vi "Host - FPGA trig export.vi"() -> ()   [LabVIEW 2019]
uses:
  <vilib>/userdefined/High Color/nirio_resource_hc.ctl
  SubVIs/Low-level/TypeDefs/TX trigger config.ctl
  FPGA/SubVIs/Utility/FPGA driver trigger source.ctl
  FPGA/SubVIs/Utility/FPGA driver trigger destination.ctl
  <vilib>/FPGAPlugInAG/PXIe-7902R/niLvFpga_Open_PXIe-7902R.vi
  <vilib>/rvi/interface/common/dynamic/niFpgaDynamicAddResources.vi
  <vilib>/Utility/error.llb/Error Cluster From Error Code.vi
  <vilib>/rvi/errors/niLvFpgaAdjustHostInterfaceError.vi
  <vilib>/FPGAPlugInAG/Dynamic/niLvFpga_Close_Dynamic.vi
  <vilib>/rvi/interface/nirviOpenFPGA/nirviOpenFPGA.xnode
  FPGA Bitfiles/barkhausenmmwave_ReceiveFPGA(3.07_FPGAtrigexport_4ZkiZJGs6ac.lvbitx
  <vilib>/rvi/interface/nirviReadWriteControl/nirviReadWriteControl.xnode
  <vilib>/rvi/interface/nirviCloseFPGA/nirviCloseFPGA.xnode
  NiFpgaLv.dll
  <vilib>/rvi/interface/Simulation/niFpgaSimulationCallBeginRW.vi
  FPGA/SubVIs/Utility/FPGA Utility.lvlib
panel:
  out "error out":T1
  in  "FPGA 2":bool
  in  "FPGA 1":bool
  in  "Trig share":T2(tab)
  in  "Sync module (export)":tag="PXI2Slot2"
  in  "Export PXI trigger":string(combo)="PXI_Trig0"
  in  "Sync module export terminal":string(combo)="PFI0"
  in  "Sync module import terminal":string(combo)="PFI0"
  in  "Import PXI trigger":string(combo)="PXI_Trig0"
  in  "Sync module (import)":tag="PXI2Slot2"
  out "fpga2.recieved PXI triggers":u16
  out "pxi0 ctr":u16
  out "pxi1 ctr":u16
  out "status":string
  in  "Stop Button":bool
  out "fpga2.recieved trigs":u16
  out "fpga1.generated trigs":u16
  in  "fpga1.trig control":bool
  in  "FPGA 2 trig":T3
  in  "FPGA 1 trig":T3
  in  "FPGA 2":T6
  in  "FPGA 1":T6
  # "MASTER"
  # "SLAVE"
  # "no trigger sharing through timing module"
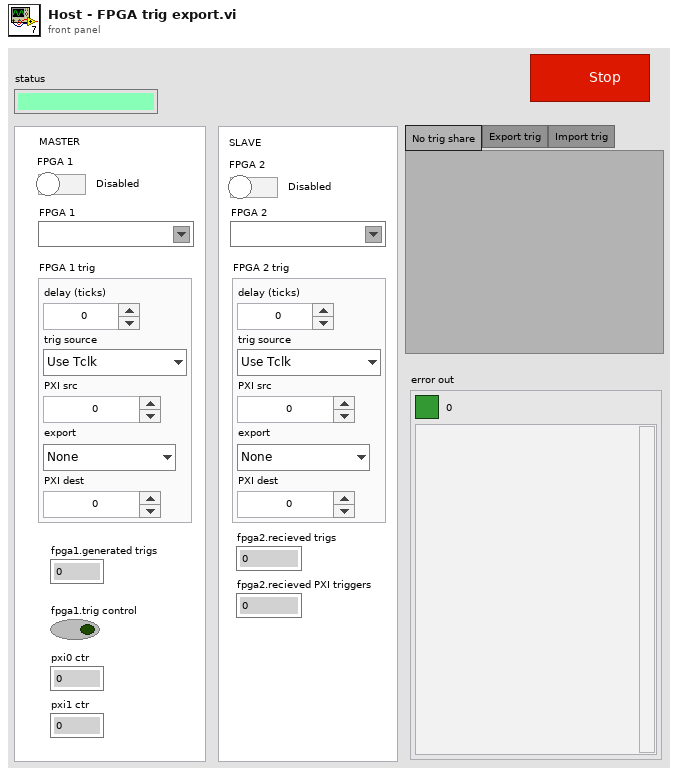
[diagram p1: front panel]
types:
  T1 = cluster{"Boolean Round":bool, "code":i32, "source":string}
  T2 = enum32{"No trig share", "Export trig", "Import trig"}
  T3 = typedef "TX trigger config.ctl" = cluster{"delay (ticks)":u16, "trig source":T4, "PXI src":i32, "export":T5, "PXI dest":i32}
  T4 = typedef "FPGA Utility.lvlib/FPGA driver trigger source.ctl" = enum16{"Use Tclk", "PXI_Trig", "Aurora RX trig"}
  T5 = typedef "FPGA Utility.lvlib/FPGA driver trigger destination.ctl" = enum16{"None", "Source trig", "Synced trig", "Delayed sync"}
  T6 = typedef "nirio_resource_hc.ctl" = tag
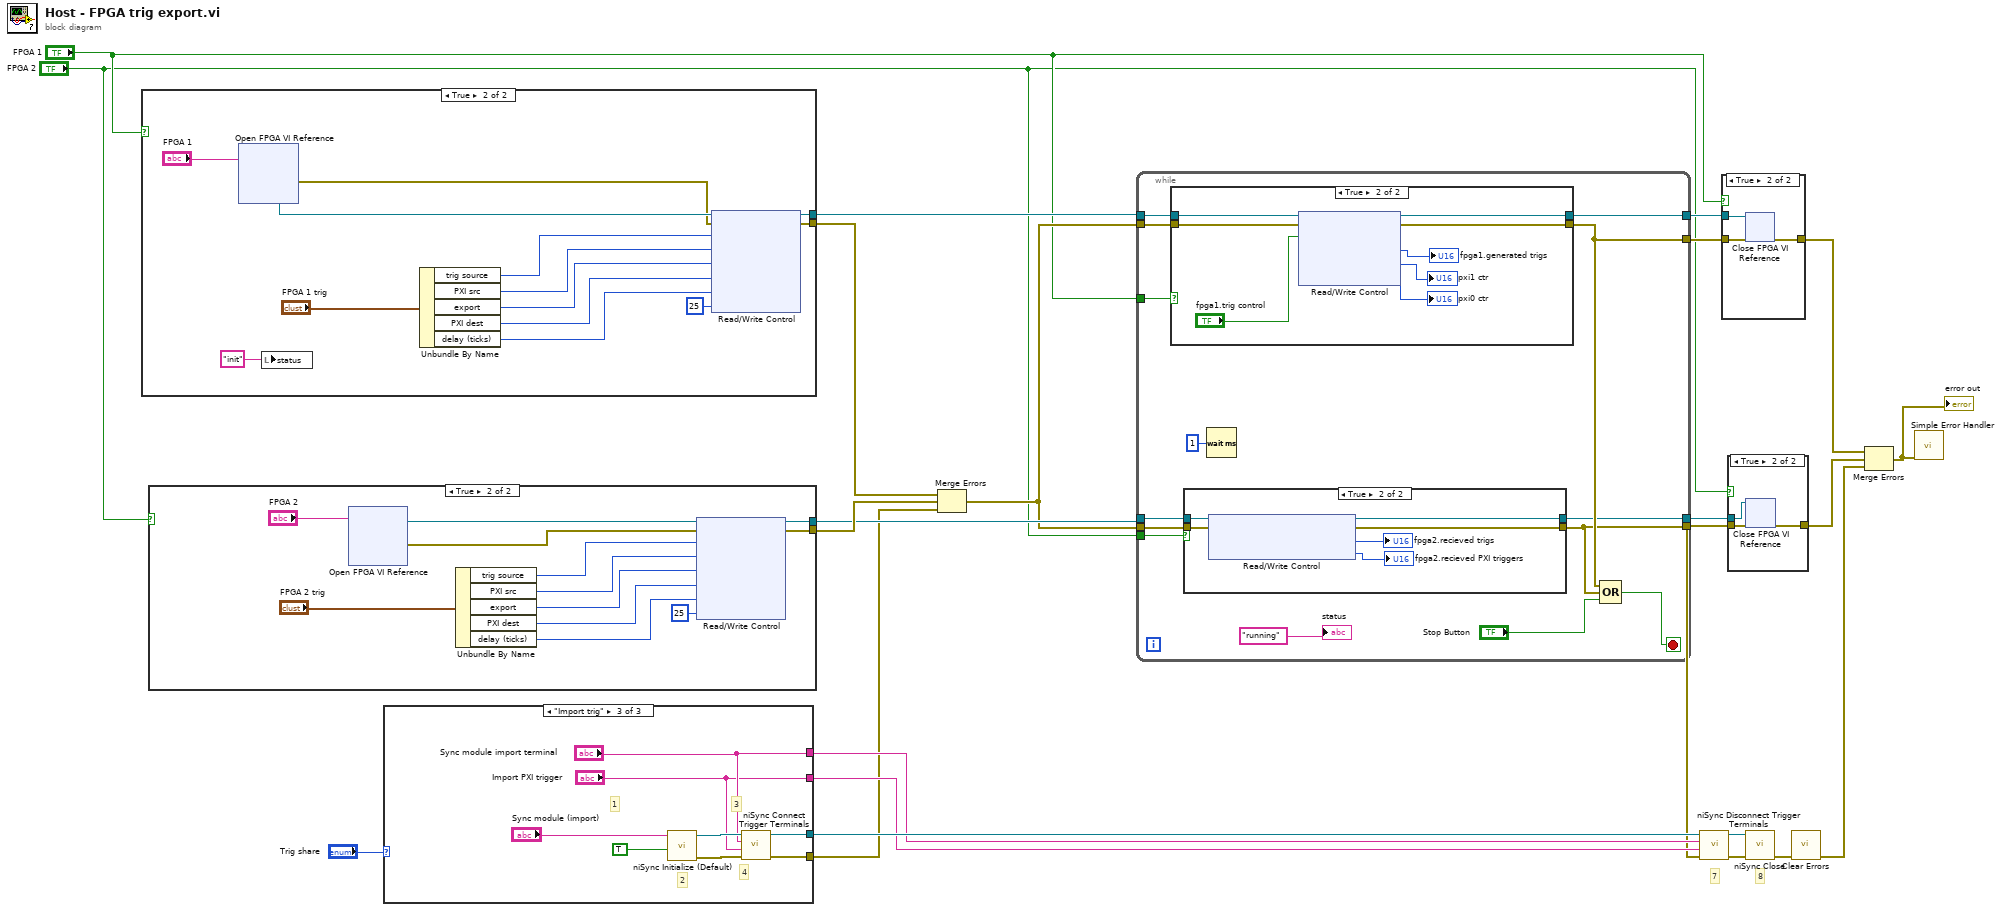
[diagram p0: block diagram]
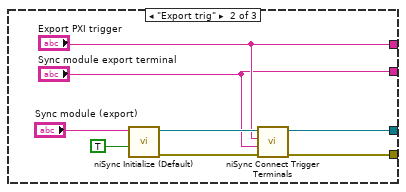
[diagram p7: hidden frame]
diagram:
  # "8"
  # "7"
  n1 = case shown="True" "FPGA 1" {
    tunnel: [_ w28] -> w22
    tunnel: [_ w27] -> w21
    frame False {
    }
    frame True {
      n2 = xnode "Open FPGA VI Reference"("resource name"="FPGA 1") -> ("FPGA VI Reference Out"=w26:refnum<k20>, "error out"=w25:errorcluster)  [unwired: 1 in]
      n3 = local write "status"("init" ("status")) -> ()
      n4 = Unbundle By Name("FPGA 1 trig") -> ("trig source"=w34:T4, "PXI src"=w33:i32, "export"=w32:T5, "PXI dest"=w31:i32, "delay (ticks)"=w30:u16)
      n5 = xnode "Read/Write Control"("FPGA VI Reference In"=w26, "error in"=w25, "trig.source"=w34, "trig.pxi src"=w33, "trig.export"=w32, "trig.pxi dst"=w31, "trig.delay"=w30, "trig.export dur"=u32 25) -> ("FPGA VI Reference Out"=w27:refnum<k20>, "error out"=w28:errorcluster)
    }
  }
  n6 = case shown="True" "FPGA 2" {
    tunnel: [_ w39] -> w23
    tunnel: [_ w38] -> w20
    frame False {
    }
    frame True {
      n7 = xnode "Open FPGA VI Reference"("resource name"="FPGA 2") -> ("FPGA VI Reference Out"=w41:refnum<k20>, "error out"=w40:errorcluster)  [unwired: 1 in]
      n8 = Unbundle By Name("FPGA 2 trig") -> ("trig source"=w42:T4, "PXI src"=w43:i32, "export"=w44:T5, "PXI dest"=w45:i32, "delay (ticks)"=w46:u16)
      n9 = xnode "Read/Write Control"("FPGA VI Reference In"=w41, "error in"=w40, "trig.source"=w42, "trig.pxi src"=w43, "trig.export"=w44, "trig.pxi dst"=w45, "trig.delay"=w46, "trig.export dur"=u32 25) -> ("FPGA VI Reference Out"=w38:refnum<k20>, "error out"=w39:errorcluster)
    }
  }
  n10 = case shown="\"Import trig\"" "Trig share" {
    tunnel: [_ w54 w59] -> w13
    tunnel: [_ "Export PXI trigger" "Sync module import terminal"] -> w10
    tunnel: [_ "Sync module export terminal" "Import PXI trigger"] -> w9
    tunnel: [_ w49 w60] -> w6
    frame "No trig share", Default {
    }
    frame "Export trig" {
      n11 = call <instrlib>:"niSync Initialize (Default).vi"("reset device (F)"=TRUE ("reset device (False)"), "resource name"="Sync module (export)") -> ("error out"=w50:errorcluster, "instrument handle out"=w56:refnum<k15>)  [unwired: 8 in]
      n12 = call <instrlib>:"niSync Connect Trigger Terminals.vi"("error in (no error)"=w50, "destination terminal"="Sync module export terminal", "source terminal"="Export PXI trigger", "instrument handle"=w56) -> ("error out"=w49:errorcluster, "instrument handle out"=w54:refnum<k15>)  [unwired: 6 in]
    }
    frame "Import trig" {
      # "4"
      # "3"
      # "2"
      # "1"
      n13 = call <instrlib>:"niSync Initialize (Default).vi"("reset device (F)"=TRUE ("reset device (False)"), "resource name"="Sync module (import)") -> ("error out"=w64:errorcluster, "instrument handle out"=w62:refnum<k15>)  [unwired: 8 in]
      n14 = call <instrlib>:"niSync Connect Trigger Terminals.vi"("error in (no error)"=w64, "destination terminal"="Import PXI trigger", "source terminal"="Sync module import terminal", "instrument handle"=w62) -> ("error out"=w60:errorcluster, "instrument handle out"=w59:refnum<k15>)  [unwired: 6 in]
    }
  }
  n15 = Merge Errors(w22, w23, w6) -> (w19:errorcluster)
  n16 = while {
    tunnel: w20 -> [w76]
    tunnel: w21 -> [w78]
    tunnel: w19 -> [w77]
    tunnel: w19 -> [w75]
    tunnel: [w72] -> w18
    tunnel: [w71] -> w17
    tunnel: [w70] -> w16
    tunnel: [w69] -> w5
    tunnel: "FPGA 1" -> [w66]
    tunnel: "FPGA 2" -> [w65]
    stop <- w73 stop-if-true
    n17 = case shown="True" w66 {
      tunnel: w78 -> [w88 w96]
      tunnel: w77 -> [w87 w95]
      tunnel: [w88 w92] -> w72
      tunnel: [w87 w91] -> w71
      frame False {
      }
      frame True {
        n18 = xnode "Read/Write Control"("FPGA VI Reference In"=w96, "error in"=w95, "trig.control"="fpga1.trig control") -> ("FPGA VI Reference Out"=w92:refnum<k20>, "error out"=w91:errorcluster, "pxi.trig dst count"=→"fpga1.generated trigs":u16, "pxi1 ctr"=→"pxi1 ctr":u16, "pxi0 ctr"=→"pxi0 ctr":u16)
      }
    }
    n19 = case shown="True" w65 {
      tunnel: w76 -> [w80 w86]
      tunnel: w75 -> [w79 w85]
      tunnel: [w80 w83] -> w70
      tunnel: [w79 w82] -> w69
      frame False {
      }
      frame True {
        n20 = xnode "Read/Write Control"("FPGA VI Reference In"=w86, "error in"=w85) -> ("FPGA VI Reference Out"=w83:refnum<k20>, "error out"=w82:errorcluster, "detected start triggers"=→"fpga2.recieved trigs":u16, "detected pxi triggers (any)"=→"fpga2.recieved PXI triggers":u16)
      }
    }
    n21 = Wait (ms)(milliseconds to wait=u32 1) -> ()  [unwired: 1 out]
    n22 = Compound Arithmetic op=OR(w71, w69, "Stop Button") -> (w73:bool)
    "status" <- "running"
  }
  n23 = call <instrlib>:"niSync Disconnect Trigger Terminals.vi"("error in (no error)"=w5, "destination terminal"=w9, "source terminal"=w10, "instrument handle"=w13) -> ("error out"=w12:errorcluster, "instrument handle out"=w11:refnum<k15>)  [unwired: 6 in]
  n24 = case shown="True" "FPGA 1" {
    tunnel: w18 -> [_ w100]
    tunnel: w17 -> [w97 w99]
    tunnel: [w97 w98] -> w14
    frame False {
    }
    frame True {
      n25 = xnode "Close FPGA VI Reference"("FPGA VI Reference In"=w100, "error in"=w99) -> ("error out"=w98:errorcluster)
    }
  }
  n26 = case shown="True" "FPGA 2" {
    tunnel: w16 -> [_ w104]
    tunnel: [w101 w103] -> w15
    tunnel: w5 -> [w101 w102]
    frame False {
    }
    frame True {
      n27 = xnode "Close FPGA VI Reference"("FPGA VI Reference In"=w104, "error in"=w102) -> ("error out"=w103:errorcluster)
    }
  }
  n28 = call <instrlib>:"niSync Close.vi"("error in (no error)"=w12, "instrument handle"=w11) -> ("error out"=w7:errorcluster)  [unwired: 9 in]
  n29 = call <vilib>:"Clear Errors.vi"("error in (no error)"=w7) -> ("error out"=w4:errorcluster)  [unwired: 5 in, 1 out]
  n30 = Merge Errors(w14, w15, w4) -> (w1:errorcluster)
  "error out" <- w1
  n31 = call <vilib>:"Simple Error Handler.vi"("error in (no error)"=w1) -> ()  [unwired: 4 in, 5 out]
